vi "Main.vi"() -> ()   [LabVIEW 2020] (continued)
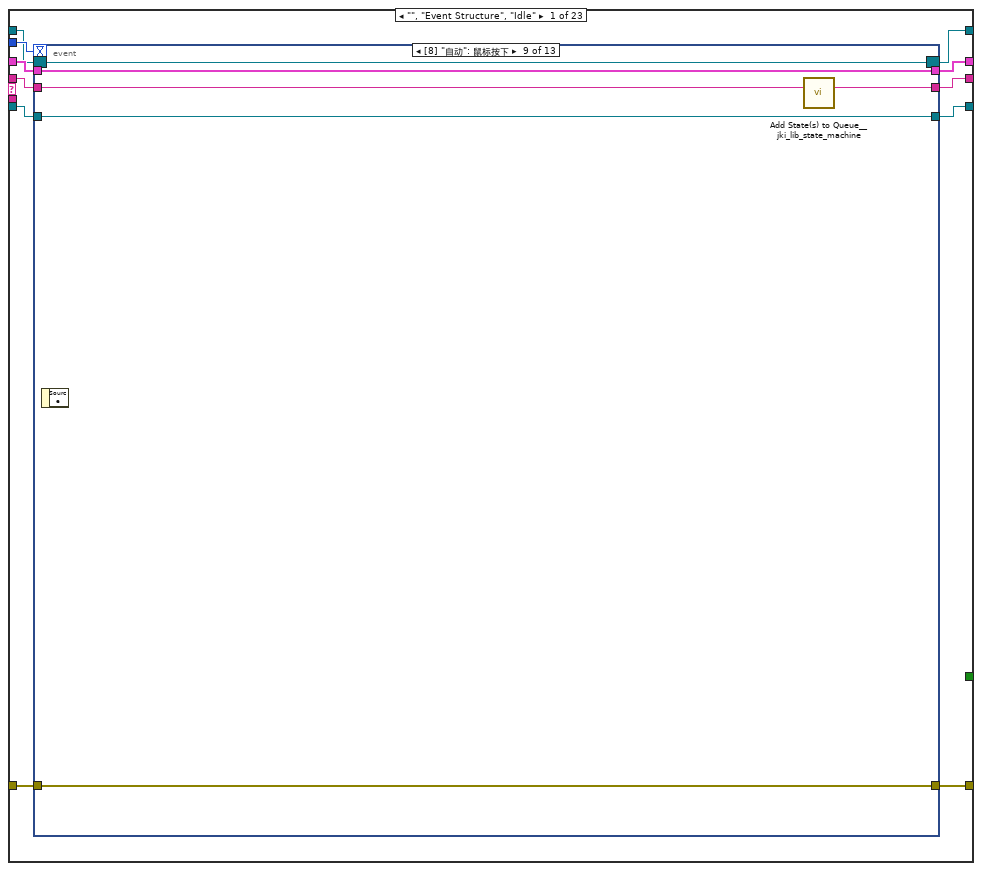
[diagram p2: hidden frame]
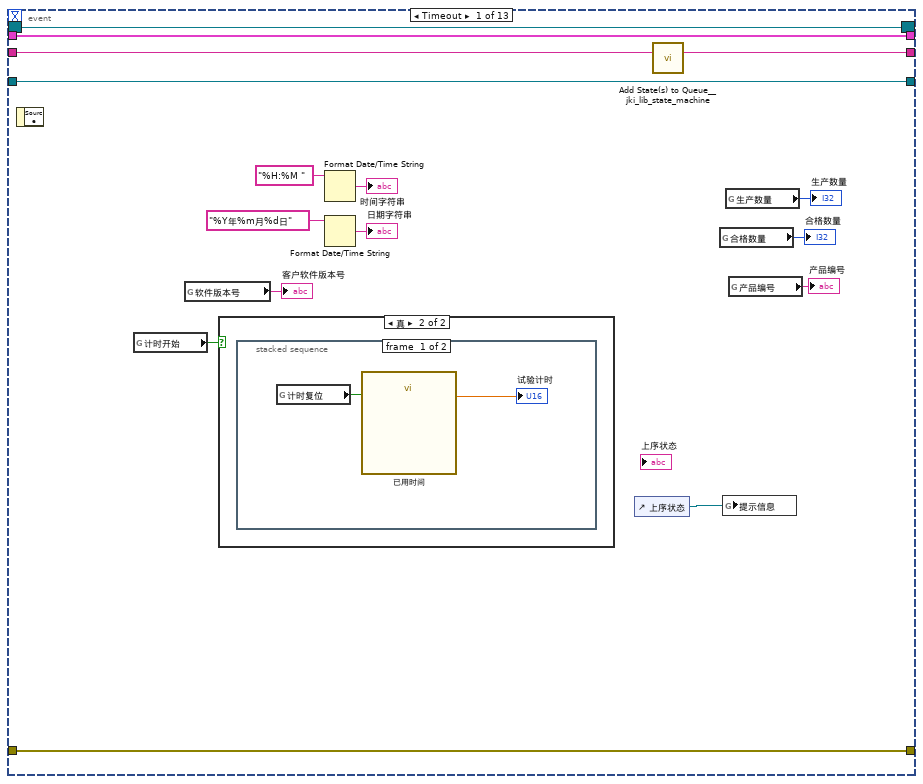
[diagram p3: hidden frame]
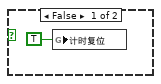
[diagram p4: hidden frame]
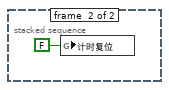
[diagram p5: hidden frame]
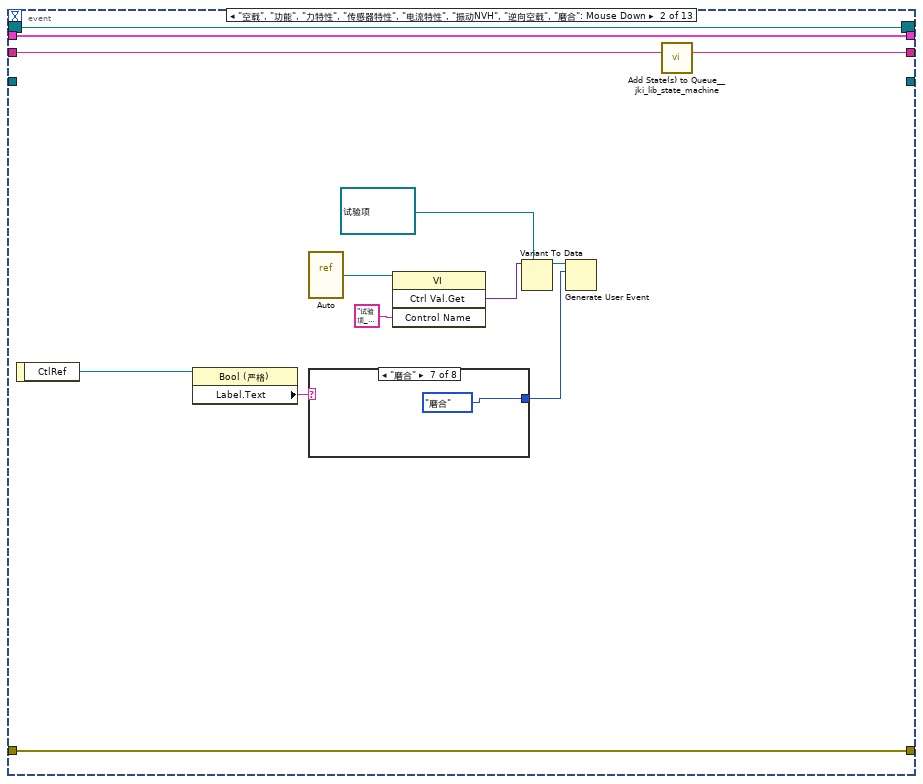
[diagram p6: hidden frame]
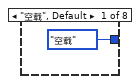
[diagram p7: hidden frame]
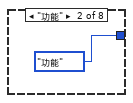
[diagram p8: hidden frame]
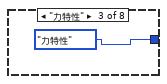
[diagram p9: hidden frame]
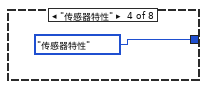
[diagram p10: hidden frame]
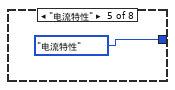
[diagram p11: hidden frame]
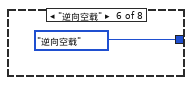
[diagram p12: hidden frame]
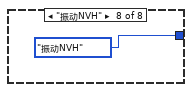
[diagram p13: hidden frame]
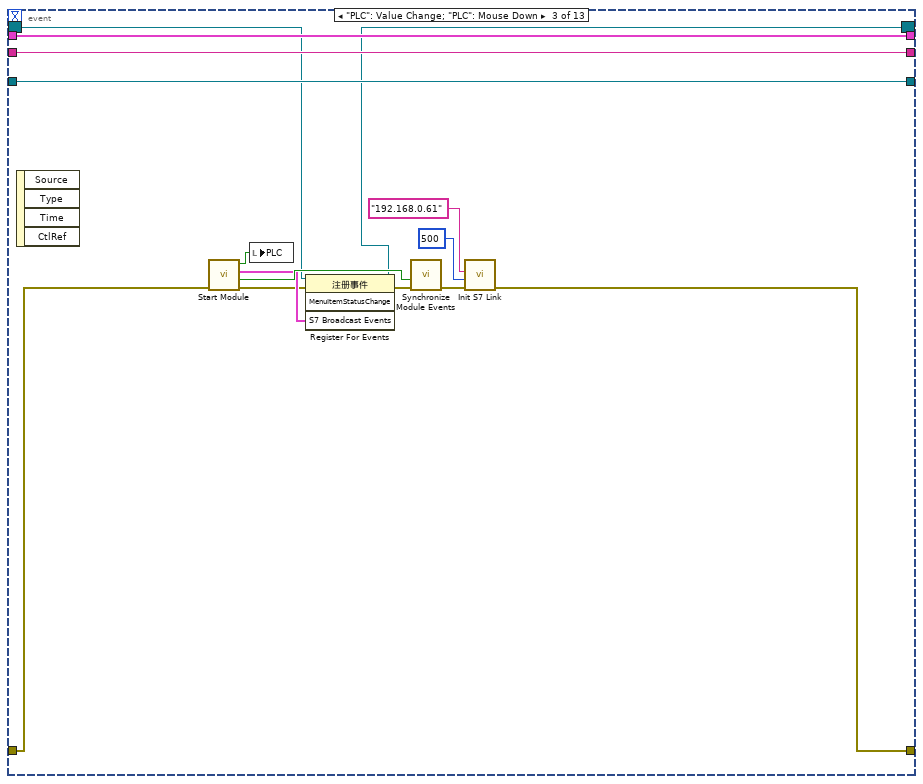
[diagram p14: hidden frame]
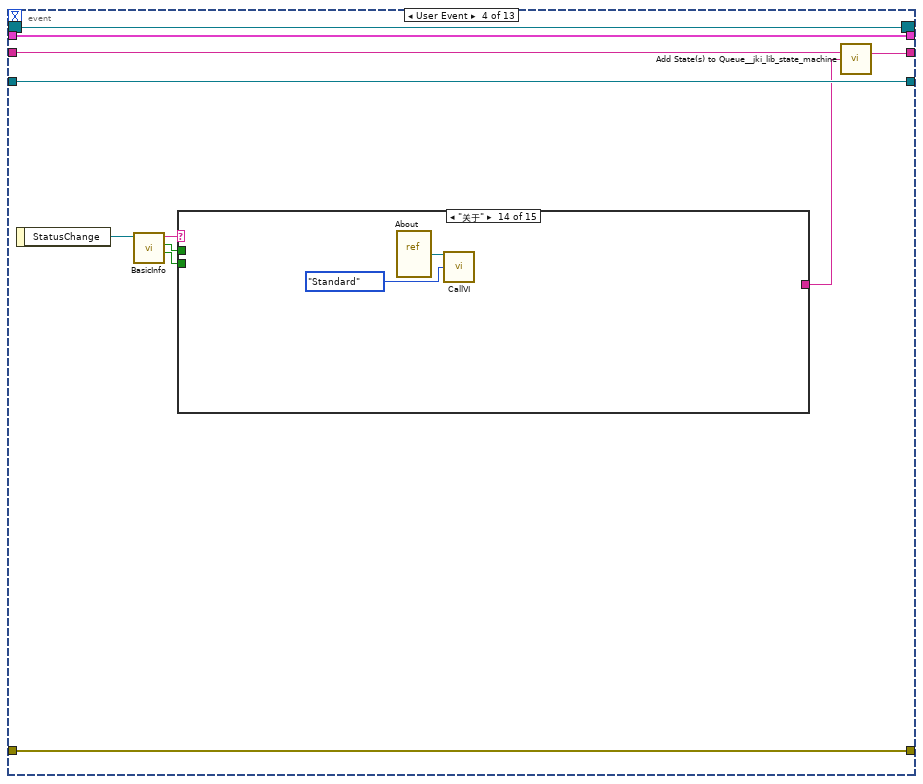
[diagram p15: hidden frame]
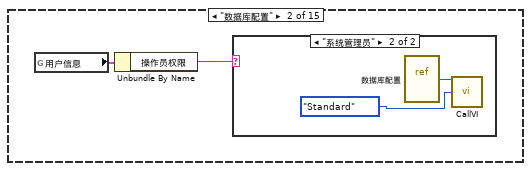
[diagram p17: hidden frame]
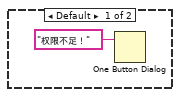
[diagram p18: hidden frame]
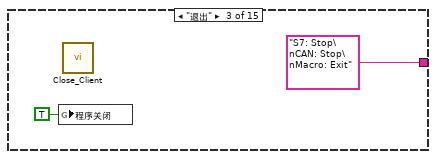
[diagram p19: hidden frame]
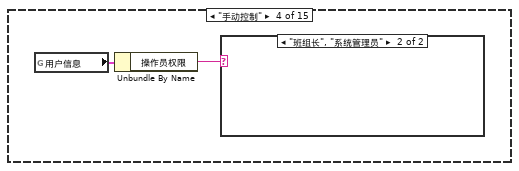
[diagram p20: hidden frame]
                    n124 = disable-structure shown="禁用" {
                      disable-tunnel: w223 -> [w225 _]
                      frame Disabled {
                        n125 = control-ref of="子面板"() -> (w224:refnum<vi>)
                        n126 = call "Call_SubPanal.vi"("VI引用句柄"=w225, "SubPnl引用句柄"=w224) -> ()  [unwired: 9 in, 1 out]
                      }
                      frame Enabled {
                      }
                    }
                    n127 = vi-ref "Auto.vi"() -> (w222:refnum<vi>)
                    n128 = invoke class="VI" method="Ctrl Val.Get"(reference=w222, "Control Name"="产品_EVENT" ("控件名")) -> ("Get Control Value Variant"=w221:variant)  [unwired: 2 in, 3 out]
                    n129 = global read "Global.vi" "产品型号"() -> (w217:string)
                    n130 = local write "产品型号"(w217) -> ()
                    n131 = Variant To Data(type=refnum<user-event> refnum ("产品_EVENT"), Variant=w221) -> (data=w218:refnum<user-event>, error out=w216:errorcluster)  [unwired: 1 in]
                    n132 = Generate User Event(user event=w218, event data cluster=w217, error in=w216) -> ()  [unwired: 1 in, 2 out]
                  }
                  frame #1 {
                    n133 = global read "Global.vi" "启用CAN"() -> (w226:bool)
                    n134 = case shown="真" w226 {
                      tunnel: ["CAN: Stop" "CAN: Stop"] -> w227
                      frame False {
                      }
                      frame True {
                        (unwired) "CAN: Stop\nIdle\nCAN: Start"
                      }
                    }
                  }
                  frame #2 {
                    n135 = control-ref of="磨合"() -> (w230:refnum<vi>)
                    n136 = control-ref of="空载"() -> (w235:refnum<vi>)
                    n137 = control-ref of="功能"() -> (w236:refnum<vi>)
                    n138 = control-ref of="力特性"() -> (w237:refnum<vi>)
                    n139 = control-ref of="电流特性"() -> (w234:refnum<vi>)
                    n140 = control-ref of="传感器特性"() -> (w233:refnum<vi>)
                    n141 = control-ref of="逆向空载"() -> (w232:refnum<vi>)
                    n142 = control-ref of="振动NVH"() -> (w231:refnum<vi>)
                    n143 = global read "Global.vi" "试验项目"() -> (w240:bool[])
                    n144 = Build Array(w235, w236, w237, w234, w233, w232, w231, w230) -> (w239:refnum<vi>[])
                    n145 = for {
                      tunnel: w239 -> [w244] mode=indexing
                      tunnel: w240 -> [w245] mode=indexing
                      shift-right: [w241] -> _
                      shift-left: 2095 -> [w242]
                      i -> [w243]
                      n146 = case shown="真" w245 {
                        tunnel: w244 -> [w246 w254]
                        tunnel: w243 -> [_ _]
                        tunnel: w242 -> [w248 w251]
                        tunnel: [w248 w249] -> w241
                        frame False {
                          n147 = property class="Bool (严格)"(reference=w246, "Top"=2000) -> ()  [unwired: 1 in, 2 out]
                        }
                        frame True {
                          n148 = Add(x=w251, y=115) -> (x+y=w249:i32)
                          n149 = Bundle(w249, 1300) -> (w252:cluster{i32, i32})  [unwired: 1 in]
                          n150 = property class="Bool (严格)"(reference=w254, "Position"=w252) -> ()  [unwired: 1 in, 2 out]
                        }
                      }
                    }
                  }
                }
              }
            }
            n151 = call <vilib>:"Add State(s) to Queue__jki_lib_state_machine.vi"("State(s) in Front (\"\")"=w207, "State(s) in (\"\")"=w210) -> ("States Out"=w211:string)  [unwired: 13 in]
          }
          event "Andon": Value Change {
            w265 = "芯轴分总成NVH" ("设备名称")
            n152 = event-data() -> ("NewVal"=w255:enum32{"未选择", "缺料报警", "质量报警", "故障报警"})  [unwired: 1 in]
            n153 = global read "用户信息.vi" "用户信息"() -> (w256:T6)
            n154 = Unbundle By Name(w256) -> ("操作员姓名"=w264:string)
            n155 = case shown="\"故障报警\"" w255 {
              tunnel: w265 -> [_ _ _ _]
              tunnel: w264 -> [_ _ _ _]
              tunnel: [enum16{"设备离线", "设备正常", "设备缺料", "设备故障", "质量报警"}."设备正常" ("设备状态") enum16{"设备离线", "设备正常", "设备缺料", "设备故障", "质量报警"}."设备缺料" ("设备状态") enum16{"设备离线", "设备正常", "设备缺料", "设备故障", "质量报警"}."质量报警" ("设备状态") enum16{"设备离线", "设备正常", "设备缺料", "设备故障", "质量报警"}."设备故障" ("设备状态")] -> w262
              frame "未选择", Default {
              }
              frame "缺料报警" {
              }
              frame "质量报警" {
              }
              frame "故障报警" {
              }
            }
            n156 = Bundle By Name(cluster=T4 {"设备名称"="", "操作人员"="", "设备状态"=enum."设备离线", "附加信息"=""} ("设备信息"), "设备名称"=w265, "操作人员"=w264, "设备状态"=w262) -> (w257:T4)
            n157 = call "Change_Client.vi"("设备信息"=w257) -> ()  [unwired: 10 in, 1 out]
          }
        }
      }
      frame "---------- Core ----------" {
        n158 = call <vilib>:"Add State(s) to Queue__jki_lib_state_machine.vi"("State(s) in (\"\")"=w275) -> ("States Out"=w274:string)  [unwired: 14 in]
      }
      frame Default {
        w287 = 42 items=["No error", "Argument error", "Memory is full", "Out of zone", "End of file", "File already open", "Generic file I/O error", "File not found", "File permission error", "Disk is full", "Duplicate path", "Too many files open", "System feature not enabled", "Resource file not found", "Cannot add resource", "Resource not found", "Image not found", "Image memory error", "Pen does not exist", "Config type invalid", "Config token not found", "Config parse error", "Config memory error", "Bad external code format", "Bad external code offset", "External code not present", "Null window", "Destroy window error", "Null menu", "Print aborted", "Bad print record", "Print driver error", "Windows error during printing", "Memory error during printing", "Print dialog error", "Generic print error", "Invalid device refnum", "Device not found", "Device parameter error", "Device unit error", "Cannot open device", "Device call aborted", "Generic error", "Cancelled by user", "Object ID too low", "Object ID too high", "Object not in heap", "Unknown heap", "Unknown object (invalid DefProc)", "Unknown object (DefProc not in table)", "Message out of range", "Invalid (null) method", "Unknown message", "Manager call not supported", "Bad address", "Network operation in progress", "Network operation timed out", "Connection is busy", "Network attribute not supported", "Network error", "Address in use", "System out of memory", "Connection aborted", "Connection refused", "Not connected", "Already connected", "Connection closed", "Initialization error (interapplication manager)", "Bad occurrence", "Wait on unbound occurrence handler", "Occurrence queue overflow", "Datalog type conflict", "Unused", "Unrecognized type (interapplication manager)", "Memory corrupt", "Failed to make temporary DLL", "Old CIN version", "Drag socket not found", "Failed to load drop-object", "Failed to register OLE object", "Failed to release OLE object", "Format specifier type mismatch", "Unknown format specifier", "Too few format specifiers", "Too many format specifiers", "Scan failed", "Newer CIN version", "Error converting to variant", "Runtime menu error", "Password tampered", "Variant attribute not found", "Incompatible variant data type", "Event data is not available", "Event Store is not present", "Occurrence is not found", "Event Queue is not created", "Event info is not available", "Refnum passed is NULL", "Error retrieving Class GUID", "Error retrieving CoClass GUID", "Error retrieving TypeLib GUID.", "Bad built application magic bytes.", "Specific driver is different from the specific driver associated with the Logical Name.", "There is no session opened to the class driver.", "Max Error", "MAX - Error with config objects", "MAX - Error loading configuration", "MAX - Group not supported"]
        # "Current State"
        n159 = Format Into String(format string="Software Exception: Unhandled State \"%s\"." ("message"), error in=w283, w278) -> (resulting string=w286:string, error out=w285:errorcluster)  [unwired: 1 in]
        n160 = call <vilib>:"Error Cluster From Error Code.vi"("show call chain? (False)"=TRUE, "error in (no error)"=w285, "error message (\"\")"=w286, "error code (0)"=w287) -> ("error out"=w284:errorcluster)  [unwired: 5 in]
        n161 = call <vilib>:"Add State(s) to Queue__jki_lib_state_machine.vi"("State(s) in (\"\")"=w282) -> ("States Out"=w281:string)  [unwired: 14 in]
      }
      frame "Initialize Core Data" {
        # "originally closed?"
        # "exe?"
        n162 = property class="VI"() -> ("Front Panel.Open"=w298:bool)  [unwired: 2 in, 2 out]
        n163 = property class="App"() -> ("App.Kind"=w297:T5)  [unwired: 2 in, 2 out]
        n164 = control-ref of="Current VI Reference"() -> (w291:refnum<vi>)
        n165 = Not(x=w298) -> (.not. x?=w295:bool)
        n166 = Equal?(x=w297, y=T5."Run Time System" ("Application:Kind")) -> (x = y?=w294:bool)
        n167 = Or(x=w295, y=w294) -> (x .or. y?=w292:bool)
        n168 = Bundle By Name(cluster=w293, "Core.Current VI Reference"=w291, "Core.Close Panel on Exit?"=w292) -> (w300:T7)
        n169 = call <vilib>:"Add State(s) to Queue__jki_lib_state_machine.vi"("State(s) in (\"\")"=w302) -> ("States Out"=w301:string)  [unwired: 14 in]
      }
      frame "Error Handler" {
        n170 = call <vilib>:"General Error Handler.vi"("error in (no error)"=w306) -> ()  [unwired: 10 in, 5 out]
        n171 = call <vilib>:"Add State(s) to Queue__jki_lib_state_machine.vi"("State(s) in Front (\"\")"="/* Post Error States", "State(s) in (\"\")"=w310) -> ("States Out"=w309:string)  [unwired: 13 in]
      }
      frame "Exit" {
        n172 = Quit LabVIEW(quit? (T)=TRUE ("退出？(T)")) -> ()
        n173 = call <vilib>:"Add State(s) to Queue__jki_lib_state_machine.vi"("State(s) in (\"\")"=w318) -> ("States Out"=w317:string)  [unwired: 14 in]
      }
      frame "--------- Library --------" {
        n174 = call <vilib>:"Add State(s) to Queue__jki_lib_state_machine.vi"("State(s) in (\"\")"=w324) -> ("States Out"=w323:string)  [unwired: 14 in]
      }
      frame "S7: Initialize" {
        n175 = property on="PLC" class="Bool (严格)"("Val(Sgnl)"=FALSE ("值(信号)")) -> ()  [unwired: 2 in, 2 out]
      }
      frame "S7: Stop" {
        n176 = call "Stop Module.vi"("error in (no error)"=w333) -> ("error out"=w332:errorcluster)  [unwired: 10 in]
        n177 = call <vilib>:"Add State(s) to Queue__jki_lib_state_machine.vi"("State(s) in (\"\")"=w334) -> ("States Out"=w335:string)  [unwired: 14 in]
      }
      frame "CAN: Start" {
        n178 = call <vilib>:"Add State(s) to Queue__jki_lib_state_machine.vi"("State(s) in (\"\")"=w340) -> ("States Out"=w341:string)  [unwired: 14 in]
      }
      frame "CAN: Stop" {
        n179 = call <vilib>:"Add State(s) to Queue__jki_lib_state_machine.vi"("State(s) in (\"\")"=w346) -> ("States Out"=w347:string)  [unwired: 14 in]
      }
      frame "---------- Data ----------" {
        n180 = call <vilib>:"Add State(s) to Queue__jki_lib_state_machine.vi"("State(s) in (\"\")"=w355) -> ("States Out"=w354:string)  [unwired: 14 in]
      }
      frame "Data: Initialize" {
        w360 = T8 {"Current VI Reference"=refnum, "Close Panel on Exit?"=FALSE}  # Core
        w362 = TRUE  # Your Boolean data
        w361 = ""  # Your string data
        n181 = global write "Global.vi" "程序关闭"(FALSE ("程序关闭")) -> ()
        n182 = global write "Global.vi" "计时开始"(FALSE ("计时结束")) -> ()
        n183 = Bundle("Core"=w360, "Your Boolean data"=w362, "Your string data"=w361) -> (w364:T7)  [unwired: 1 in]
        n184 = call <vilib>:"Add State(s) to Queue__jki_lib_state_machine.vi"("State(s) in (\"\")"=w366) -> ("States Out"=w365:string)  [unwired: 14 in]
      }
      frame "Data: Cleanup" {
        n185 = Unbundle By Name(w369) -> ("Core.Current VI Reference"=w372:refnum<vi>)
        n186 = Close Reference(reference=w372, error in (no error)=w371) -> (error out=w370:errorcluster)
        n187 = call <vilib>:"Add State(s) to Queue__jki_lib_state_machine.vi"("State(s) in (\"\")"=w374) -> ("States Out"=w373:string)  [unwired: 14 in]
      }
      frame "---------- UI ----------" {
        # "Do not put any code in this frame.\n(It is a separator no-op. You can make a copy of this frame to create a new UI frame)"
        n188 = call <vilib>:"Add State(s) to Queue__jki_lib_state_machine.vi"("State(s) in (\"\")"=w380) -> ("States Out"=w379:string)  [unwired: 14 in]
      }
      frame "UI: Initialize" {
        n189 = disable-structure shown="启用" {
          disable-tunnel: [w394 _] -> w384
          disable-tunnel: w381 -> [w392 _]
          frame Enabled {
            n190 = vi-ref "Auto.vi"() -> (w393:refnum<vi>)
            n191 = property class="VI"(reference=w393) -> (reference out=w391:refnum<vi>, "FP.State"=w390:T3)  [unwired: 1 in, 1 out]
            n192 = case shown="\"Invalid\", \"Closed\"" w390 {
              tunnel: w392 -> [w400 w402]
              tunnel: w391 -> [w401 w403]
              tunnel: [w399 w403] -> w388
              tunnel: [w398 w402] -> w389
              frame "Standard", Default {
                n193 = invoke class="VI" method="FP.Close"(reference=w401, error in=w400) -> (reference out=w399:refnum<vi>, error out=w398:errorcluster)  [unwired: 1 in, 1 out]
              }
              frame "Invalid", "Closed" {
              }
            }
            n194 = invoke on="子面板" class="SubPnl" method="Insert VI"(error in=w389, "VI Ref"=w388) -> (error out=w397:errorcluster)  [unwired: 2 in, 3 out]
            n195 = invoke class="VI" method="Run VI"(reference=w388, error in=w397, "Wait until done"=FALSE ("结束前等待"), "Auto Dispose Ref"=TRUE ("自动销毁引用")) -> (error out=w394:errorcluster)  [unwired: 1 in, 4 out]
          }
          frame Disabled {
            n196 = vi-ref "Auto.vi"() -> (w405:refnum<vi>)
            n197 = call "CallVI.vi"("VI引用"=w405, "状态"=T3."Maximized") -> ()  [unwired: 12 in, 2 out]
          }
        }
        n198 = call <vilib>:"Add State(s) to Queue__jki_lib_state_machine.vi"("State(s) in (\"\")"=w387) -> ("States Out"=w386:string)  [unwired: 14 in]
      }
      frame "UI: Init" {
        n199 = stacked-sequence {
          tunnel: w407 -> [_ _ _ _ _]
          frame #0 {
            n200 = vi-ref "传感器读取.vi"() -> (w413:refnum<vi>)
            n201 = disable-structure shown="禁用" {
              frame Disabled {
                n202 = call "Open.vi"() -> ()  [unwired: 11 in, 1 out]
              }
              frame Enabled {
              }
            }
            n203 = call "CallVI.vi"("VI引用"=w413, "状态"=T3."Hidden") -> ()  [unwired: 12 in, 2 out]
          }
          frame #1 {
            n204 = global write "Global.vi" "程序关闭"(FALSE ("程序关闭")) -> ()
            n205 = control-ref of="电流特性"() -> (w418:refnum<vi>)
            n206 = control-ref of="空载"() -> (w421:refnum<vi>)
            n207 = control-ref of="力特性"() -> (w419:refnum<vi>)
            n208 = control-ref of="功能"() -> (w420:refnum<vi>)
            n209 = global write "A180648.vi" "LED-电流特性"(w418) -> ()
            n210 = global write "A180648.vi" "LED-空载"(w421) -> ()
            n211 = global write "A180648.vi" "LED-力特性"(w419) -> ()
            n212 = global write "A180648.vi" "LED-功能"(w420) -> ()
            n213 = control-ref of="逆向空载"() -> (w417:refnum<vi>)
            n214 = control-ref of="振动NVH"() -> (w415:refnum<vi>)
            n215 = control-ref of="磨合"() -> (w414:refnum<vi>)
            n216 = control-ref of="传感器特性"() -> (w416:refnum<vi>)
            n217 = global write "A180648.vi" "LED-传感器特性"(w416) -> ()
            n218 = global write "A180648.vi" "LED-逆向空载"(w417) -> ()
            n219 = global write "A180648.vi" "LED-振动NVH"(w415) -> ()
            n220 = global write "A180648.vi" "LED-磨合"(w414) -> ()
          }
          frame #2 {
            w429 = 0
            n221 = shared-variable "我的电脑\\Global.lvlib\\总成追溯码"("   " ("工位追溯码")) -> ()  [unwired: 1 in, 1 out]
            n222 = global write "Global.vi" "生产数量"(w429) -> ()
            n223 = global write "Global.vi" "合格数量"(w429) -> ()
            n224 = global read "Global.vi" "用户信息"() -> (w426:T9)
            n225 = global read "Global.vi" "联机模式"() -> (w423:enum16{"单机", "追溯"})
            n226 = Unbundle By Name(w426) -> ("用户名"=→"userName":string, "用户权限"=→"userStatus":string)
            n227 = case shown="\"追溯\"" w423 {
              tunnel: ["联网" ("connectionMode") "单机" ("connectionMode")] -> w430
              frame "追溯" {
              }
              frame "单机", Default {
              }
            }
            "connectionMode" <- w430
            "产品型号" <- "" ("产品型号")
          }
          frame #3 {
            n228 = control-ref of="提示信息"() -> (w434:refnum<vi>)
            n229 = control-ref of="自动"() -> (w435:refnum<vi>)
            n230 = control-ref of="错误"() -> (w436:refnum<vi>)
            n231 = control-ref of="Result"() -> (w437:refnum<vi>)
            n232 = control-ref of="更换产品"() -> (w433:refnum<vi>)
            n233 = global write "Global.vi" "提示信息"(w434) -> ()
            n234 = global write "Global.vi" "程序自动"(w435) -> ()
            n235 = global write "Global.vi" "报警图标"(w436) -> ()
            n236 = global write "Global.vi" "Result"(w437) -> ()
            n237 = global write "Global.vi" "更换产品"(w433) -> ()
          }
          frame #4 {
            n238 = global read "Global.vi" "Result"() -> (w440:refnum<vi>)
            n239 = property class="Tbl"(reference=w440, "Row Headers[]"=string[] [], "Value"=string[][] []) -> ()  [unwired: 1 in, 2 out]
            n240 = disable-structure shown="禁用" {
              frame Disabled {
                n241 = call "Start_Client.vi"() -> ()  [unwired: 12 in]
              }
              frame Enabled {
              }
            }
          }
        }
        n242 = call <vilib>:"Add State(s) to Queue__jki_lib_state_machine.vi"("State(s) in (\"\")"=w411) -> ("States Out"=w410:string)  [unwired: 14 in]
      }
      frame "UI: Config" {
        n243 = vi-ref "Config.vi"() -> (w443:refnum<vi>)
        n244 = call "CallVI.vi"("VI引用"=w443, "状态"=T3."Standard") -> ()  [unwired: 12 in, 2 out]
        n245 = call <vilib>:"Add State(s) to Queue__jki_lib_state_machine.vi"("State(s) in (\"\")"=w448) -> ("States Out"=w447:string)  [unwired: 14 in]
      }
      frame "UI: Cursor Set" {
        # "Argument"
        n246 = case shown="\"Idle\", 默认" w451 {
          tunnel: w453 -> [w458 w460]
          tunnel: [w457 w459] -> w452
          frame "Idle", Default {
            n247 = call <vilib>:"Unset Busy.vi"("error in (no error)"=w458) -> ("error out"=w457:errorcluster)  [unwired: 10 in]
          }
          frame "Busy" {
            n248 = call <vilib>:"Set Busy.vi"("error in (no error)"=w460) -> ("error out"=w459:errorcluster)  [unwired: 9 in, 1 out]
          }
        }
        n249 = call <vilib>:"Add State(s) to Queue__jki_lib_state_machine.vi"("State(s) in (\"\")"=w456) -> ("States Out"=w455:string)  [unwired: 14 in]
      }
      frame "UI: Front Panel State" {
        # "Argument"
        n250 = Unbundle By Name(w465) -> ("Core.Current VI Reference"=w464:refnum<vi>)
        n251 = case shown="\"Close\"" w463 {
          tunnel: w467 -> [w473 w486]
          tunnel: [w475 w487] -> w466
          tunnel: w464 -> [w474 w484]
          frame "Open", Default {
            n252 = property class="VI"(reference=w474, error in=w473) -> (reference out=w471:refnum<vi>, error out=w472:errorcluster, "Front Panel.Open"=w470:bool)
            n253 = case shown="假" w470 {
              tunnel: [w478 w481] -> w475
              tunnel: w472 -> [w477 w481]
              tunnel: w471 -> [w476 _]
              frame False {
                n254 = invoke class="VI" method="FP.Open"(reference=w476, error in=w477, "Activate"=TRUE, "State"=T3."Standard") -> (error out=w478:errorcluster)  [unwired: 1 in, 4 out]
              }
              frame True {
              }
            }
          }
          frame "Close" {
            n255 = property class="VI"(reference=w484, error in=w486) -> (reference out=w483:refnum<vi>, error out=w485:errorcluster, "Front Panel.Open"=w482:bool)
            n256 = case shown="真" w482 {
              tunnel: [w488 w491] -> w487
              tunnel: w485 -> [w488 w490]
              tunnel: w483 -> [_ w489]
              frame False {
              }
              frame True {
                n257 = invoke class="VI" method="FP.Close"(reference=w489, error in=w490) -> (error out=w491:errorcluster)  [unwired: 1 in, 2 out]
              }
            }
          }
        }
        n258 = call <vilib>:"Add State(s) to Queue__jki_lib_state_machine.vi"("State(s) in (\"\")"=w469) -> ("States Out"=w468:string)  [unwired: 14 in]
      }
      frame "---------- Macro ----------" {
        n259 = call <vilib>:"Add State(s) to Queue__jki_lib_state_machine.vi"("State(s) in (\"\")"=w497) -> ("States Out"=w496:string)  [unwired: 14 in]
      }
      frame "Macro: Initialize" {
        n260 = call <vilib>:"Add State(s) to Queue__jki_lib_state_machine.vi"("State(s) in Front (\"\")"="Data: Initialize\nInitialize Core Data\nS7: Initialize\nIdle\nUI: Init\nUI: Front Panel State >> Open\nUI: Initialize\nUI: Config", "State(s) in (\"\")"=w504) -> ("States Out"=w503:string)  [unwired: 13 in]
      }
      frame "Macro: Exit" {
        n261 = Unbundle By Name(w514) -> ("Core.Close Panel on Exit?"=w513:bool)
        n262 = Quit LabVIEW(quit? (T)=TRUE ("退出？(T)")) -> ()
        n263 = Select(t="UI: Front Panel State >> Close", s=w513, f="") -> (s? t:f=w510:string)
        n264 = call <vilib>:"Add State(s) to Queue__jki_lib_state_machine.vi"("State(s) in (\"\")"=w510, "State(s) at Back (\"\")"="Data: Cleanup\nExit") -> ("States Out"=w508:string)  [unwired: 13 in]
        n265 = call <vilib>:"Add State(s) to Queue__jki_lib_state_machine.vi"("State(s) in Front (\"\")"=w508, "State(s) in (\"\")"=w517) -> ("States Out"=w516:string)  [unwired: 13 in]
      }
    }
  }
  n266 = call-dynamic "Cleanup.vi"("MenuStrip in"=w6) -> ()  [unwired: 10 in, 1 out]
